vi "labHolo.vi"() -> ()   [LabVIEW 2023] (continued)
    tunnel: [w306] -> w9
    tunnel: w7 -> [w304]
    tunnel: w5 -> [w323]
    tunnel: w4 -> [w303]
    tunnel: w3 -> [w302]
    tunnel: w14 -> [w1060]
    tunnel: w12 -> [w1057]
    tunnel: w11 -> [w1056]
    tunnel: w10 -> [w1055]
    tunnel: w9 -> [w1054]
    frame #0 {
      w66 = T15 7 items=["Grayscale (U8)", "Grayscale (I16)", "Grayscale (SGL)", "Complex (CSG)", "RGB (U32)", "HSL (U32)", "RGB (U64)", "Grayscale (U16)"] ("Image Type")
      w68 = T15 4 items=["Grayscale (U8)", "Grayscale (I16)", "Grayscale (SGL)", "Complex (CSG)", "RGB (U32)", "HSL (U32)", "RGB (U64)", "Grayscale (U16)"] ("Image Type")
      # "Controls definition"
      n2 = Current VI's Path() -> (path=w133:path)
      n3 = Strip Path(path=w133) -> (stripped path=→"path":path)  [unwired: 1 out]
      n4 = case shown="\"16bits\", Default" "bit depth" {
        tunnel: [w152 w154] -> w117
        tunnel: [TRUE FALSE] -> w122
        frame "16bits", Default {
          w152 = T15 7 items=["Grayscale (U8)", "Grayscale (I16)", "Grayscale (SGL)", "Complex (CSG)", "RGB (U32)", "HSL (U32)", "RGB (U64)", "Grayscale (U16)"] ("Image Type")
        }
        frame "8bits" {
          w154 = T15 0 items=["Grayscale (U8)", "Grayscale (I16)", "Grayscale (SGL)", "Complex (CSG)", "RGB (U32)", "HSL (U32)", "RGB (U64)", "Grayscale (U16)"] ("Image Type")
        }
      }
      n5 = call "IMAQ Create"("Image Name"="monoHolo", "Image Type"=w66) -> ("New Image"=w65:T6)  [unwired: 3 in, 1 out]
      n6 = call "labHolo_path.vi"("sub folder or file (str)"="SupportFiles\\TestPatterns\\no_image.png") -> ("labHolo path"=w98:path)  [unwired: 1 in, 1 out]
      n7 = call "IMAQ Create"("Image Name"="holoSLM", "Image Type"=w68) -> ("New Image"=w63:T6)  [unwired: 3 in, 1 out]
      n8 = call "IMAQ Create"("Image Name"="holoMonitor", "Image Type"=w68) -> ("New Image"=w64:T6, "error out"=w67:errorcluster)  [unwired: 3 in]
      n9 = call "IMAQ Create"("Image Name"="Theo. beam", "Image Type"=w68) -> ("New Image"=w93:T6)  [unwired: 3 in, 1 out]
      n10 = call "positionManager.vi"("Display"=2, "Cluster"="2_posCluster") -> ("output cluster"=w107:cluster{i32, i32})  [unwired: 5 in, 2 out]
      n11 = call "positionManager.vi"("Display"=1, "Cluster"="1_posCluster") -> ("output cluster"=w106:cluster{i32, i32})  [unwired: 5 in, 2 out]
      n12 = call "initialize.vi"("14bits"=w122, "sys Python version"="3.9") -> ("session out"=w61:refnum<k35>, "available cameras"=w129:cluster{string[], string[]}, "error out"=w128:errorcluster)  [unwired: 2 in]
      "available\ncameras" <- w129
      n13 = case shown="1" "SLM_number" {
        tunnel: [w144 w146] -> w112
        tunnel: [w143 w148] -> w111
        tunnel: "1_posCluster" -> [w144 _]
        tunnel: "1_mainPos" -> [w143 _]
        tunnel: "2_posCluster" -> [_ w146]
        tunnel: "2_mainPos" -> [_ w148]
        tunnel: "SLM1 cluster" -> [w142 _]
        tunnel: "SLM2 cluster" -> [_ w147]
        tunnel: [w142 w147] -> w100
        tunnel: [w141 w145] -> w101
        tunnel: w107 -> [_ w145]
        tunnel: w106 -> [w141 _]
        frame 0, Default {
        }
        frame 1 {
        }
      }
      n14 = Unbundle(w129) -> (w114:string[])  [unwired: 1 out]
      n15 = local read "Selected Newport Device"() -> (w78:T1)
      n16 = call "IMAQ Create"("Image Name"="ROI image", "Image Type"=w117) -> ("New Image"=w116:T6)  [unwired: 3 in, 1 out]
      n17 = call "IMAQ Create"("Image Name"="Ref Image", "Image Type"=w117) -> ("New Image"=w119:T6)  [unwired: 3 in, 1 out]
      n18 = call "IMAQ Create"("Image Name"="CCD Image", "Image Type"=w117) -> ("New Image"=w120:T6)  [unwired: 3 in, 1 out]
      n19 = property on="Camera ID" class="Ring (strict)"("Strings []"=w114) -> ("Value"=w90:u16)  [unwired: 2 in, 2 out]
      n20 = Open Python Session(python version="3.9") -> (session out=w60:refnum<k35>)  [unwired: 2 in, 1 out]
      n21 = call "Connect Newport Instrument.vi"("Selected Device Cluster (INPUT)"=w78) -> ("error (duplicate)"=w77:errorcluster, "Device Connection Cluster"=w75:T16, "Selected Device Cluster (OUTPUT)"=w74:T1)  [unwired: 5 in, 3 out]
      n22 = property on="Zoom2Fit" class="Bool (strict)"("DisabledEnum"=T10."Disabled and Grayed Out" ("Disabled")) -> ()  [unwired: 2 in, 2 out]
      n23 = Bundle("New Image"=w65, "New Image"=w64, "New Image"=w63) -> (w62:T17)  [unwired: 1 in]
      n24 = Unbundle(w101) -> (→"Xpos":i32, →"Ypos":i32)
      n25 = Array Size(array=w114) -> (size(s)=w84:i32)
      n26 = case shown="No Error" w77 {
        tunnel: [w137 w140] -> w76
        tunnel: w75 -> [w137 _]
        tunnel: w74 -> [w136 _]
        tunnel: [w136 w138] -> w73
        frame No Error {
        }
        frame Error {
          n27 = call "Connect Newport Instrument.vi"("Selected Device Cluster (INPUT)"=T11 {"Found resources names"=["ASRL1::INSTR", "ASRL3::INSTR"], "Found interfaces names"=["ASRL1  (COM1 - Puerto de comunicaciones)", "ASRL3  (COM3 - USB Serial Port)"], "OK?"=FALSE, "Selected device"="", "Address"=0, "error"={"status"=TRUE, "code"=0, "source"=""}}) -> ("Device Connection Cluster"=w140:T16, "Selected Device Cluster (OUTPUT)"=w138:T1)  [unwired: 5 in, 4 out]
        }
      }
      "Selected Newport Device" <- w73
      n28 = Index Array(array=w114, index=0) -> (element=w115:string)
      n29 = local write "EnlargeCCD"(FALSE) -> ()
      n30 = case shown="\"Any\", Default" w115 {
        tunnel: w90 -> [_ _]
        tunnel: [FALSE TRUE] -> w89
        frame "Any", Default {
        }
        frame "NotFound" {
        }
      }
      n31 = call "rearrengeArray.vi"("array in"="exposures", "desired size"=w84) -> ("array out"=w82:dbl[])
      n32 = Not(x="Devel?") -> (.not. x?=w87:bool)
      n33 = call "rearrengeArray.vi"("array in"="FPSs", "desired size"=w84) -> ("array out"=w85:dbl[])
    }
    frame #1 {
      w187 = FALSE ("Visible")
      # "just in case, no image"
      # "CHANGE THIS!"
      # "Indicators (setting up)"
      n34 = And(x=w207, y=w206) -> (x .and. y?=w208:bool)
      n35 = Unbundle By Name(w248) -> ("1_Xcenter"=→"Xcenter":dbl, "1_Ycenter"=→"Ycenter":dbl, "1_Diam. X"=→"Diam. X":dbl, "1_Diam. Y"=→"Diam. Y":dbl, "1_Form fa."=→"Form fa.":dbl)
      n36 = for {
        N: w203 -> [_]
        tunnel: w222 -> [w289]
        tunnel: w221 -> [w288]
        tunnel: [w287] -> w220
        tunnel: [w286] -> w216 mode=indexing
        tunnel: [w285] -> w217 mode=indexing
        tunnel: [w283] -> w214 mode=indexing
        tunnel: [w282] -> w213
        tunnel: w211 -> [w281] mode=indexing
        tunnel: w212 -> [w280] mode=indexing
        tunnel: w207 -> [w276]
        i -> [w279]
        n37 = call "start.vi"("Not found"=w276, "Cam id"=w279, "error in (no error)"=w288, "Exposure (ms)"=w280, "FPS"=w281, "session in"=w289) -> ("error out"=w282:errorcluster, "cam attr."=w284:T18, "session out"=w287:refnum<k35>)  [unwired: 2 in]
        n38 = Unbundle By Name(w284) -> ("x"=w278:i32, "y"=w277:i32, "FPS"=w286:dbl, "Exposure"=w285:dbl)
        n39 = Bundle("x"=w278, "y"=w277) -> (w283:cluster{"x":i32, "y":i32})  [unwired: 1 in]
      }
      "Cam sizes" <- w214
      n40 = Unbundle By Name(w247) -> ("1_Xoffset"=w257:dbl, "1_Yoffset"=w256:dbl, "1_Xgros"=w255:dbl, "1_Ygros"=w254:dbl, "1_Xfine"=w253:dbl, "1_Yfine"=w252:dbl, "1_Xreverse"=w251:u16, "1_Yreverse"=w250:u16, "1_XYswap"=w249:u16)
      n41 = Increment(x=w201) -> (x+1=w202:u16)
      n42 = Unbundle By Name(w231) -> ("1_Radio"=w182:T7, "1_Trans"=w246:dbl, "1_Phase"=w245:dbl, "1_HoloCode"=w244:string, "1_Semi"=w243:bool, "1_Active"=w242:u16, "1_ModType"=w241:string, "1_Flip"=w240:string, "1_HoloNum"=w239:dbl, "1_key1"=w238:string, "1_value1"=w237:i64, "1_key2"=w236:string, "1_value2"=w159:i64, "1_Calibration file"=w158:string, "1_SLM brand"=w157:string)
      n43 = case shown="False" w208 {
        tunnel: [T10."Enabled" ("Disabled") T10."Disabled and Grayed Out" ("Disabled")] -> w200
        frame False {
        }
        frame True {
        }
      }
      n44 = Greater?(x=w202, y=w203) -> (0:w204:bool)
      n45 = call "CONEX-CC Get Stage Identifier v2.vi"("Connection Cluster in"=w194) -> ("Identifier"=→"ID":string, "Connection Cluster out"=w190:T16)  [unwired: 9 in]
      n46 = call "IMAQ ReadFile"("File Path"=w175, "Image"=w263) -> ("Image Out"=w262:T6)  [unwired: 5 in, 4 out]
      n47 = case shown="0, Default" w233 {
        tunnel: [u16 2 u16 1] -> w181
        tunnel: [u16 1 ("Display") u16 2 ("Display")] -> w174
        tunnel: [w293 w301] -> w172
        tunnel: w173 -> [w293 w300]
        tunnel: w171 -> [w292 w301]
        tunnel: [w292 w300] -> w156
        tunnel: [w291 w297] -> w163
        tunnel: w162 -> [w290 w297]
        tunnel: w161 -> [w291 w296]
        tunnel: [w290 w296] -> w160
        frame 0, Default {
        }
        frame 1 {
        }
      }
      n48 = property on="FPS" class="DigNum (strict)"("DisabledEnum"=w200) -> ()  [unwired: 2 in, 2 out]
      n49 = property on="bit depth" class="Enum (strict)"("DisabledEnum"=w200) -> ()  [unwired: 2 in, 2 out]
      n50 = property on="Gain" class="DigNum (strict)"("DisabledEnum"=w200) -> ()  [unwired: 2 in, 2 out]
      n51 = call "getSavePath.vi"("beam_name"=w226, "Polarizer"=w225, "Analyzer"=w224, "prefix"=w223, "suffix"=w264, "active"=w186) -> ("appended filename"=→"default filename":string)  [unwired: 9 in]
      n52 = property on="(1) Go to:" class="DigNum (strict)"("Caption.Text"=w196) -> ()  [unwired: 2 in, 2 out]
      n53 = property on="(2) Go to:" class="DigNum (strict)"("Caption.Text"=w196) -> ()  [unwired: 2 in, 2 out]
      n54 = property on="Step:" class="DigNum (strict)"("Caption.Text"=w196) -> ()  [unwired: 2 in, 2 out]
      n55 = property on="Raw position" class="DigNum (strict)"("Caption.Text"=w196) -> ()  [unwired: 2 in, 2 out]
      n56 = property on="Relative pos." class="DigNum (strict)"("Caption.Text"=w196) -> ()  [unwired: 2 in, 2 out]
      n57 = property on="Zero pos." class="DigNum (strict)"("Caption.Text"=w196) -> ()  [unwired: 2 in, 2 out]
      n58 = local write "Gain"(0.0 ("Gain")) -> ()
      n59 = case shown="False" w204 {
        frame False {
        }
        frame True {
          n60 = local write "Camera ID"(u16 0) -> ()
        }
      }
      n61 = local write "Xreverse"(w251) -> ()
      n62 = local write "Yreverse"(w250) -> ()
      n63 = local write "XYswap"(w249) -> ()
      n64 = local write "Xoffset"(w257) -> ()
      n65 = local write "Ygros"(w254) -> ()
      n66 = local write "Xfine"(w253) -> ()
      n67 = local write "Yoffset"(w256) -> ()
      n68 = local write "Xgros"(w255) -> ()
      n69 = local write "Yfine"(w252) -> ()
      n70 = property on="stop travel" class="Bool (strict)"("Visible"=w187, "Value"=w187) -> ()  [unwired: 2 in, 2 out]
      n71 = call "loadShowHolo.vi"("mainPos"=w160, "Python session"=w176, "Display"=w181, "error in (no error)"=w180, "prev. path"=w175, "SLM1 cluster"=w172, "holoImages"=w169) -> ("error out"=w177:errorcluster)  [unwired: 1 in, 3 out]
      n72 = property on="Exposure (ms)" class="DigNum (strict)"("DisabledEnum"=w200) -> ()  [unwired: 2 in, 2 out]
      n73 = property on="Camera ID" class="Ring (strict)"("DisabledEnum"=w200) -> ()  [unwired: 2 in, 2 out]
      n74 = local write "Radio"(w182) -> ()
      n75 = local write "Trans"(w246) -> ()
      n76 = local write "Phase"(w245) -> ()
      n77 = local write "HoloCode"(w244) -> ()
      n78 = local write "Semi"(w243) -> ()
      n79 = local write "Active"(w242) -> ()
      n80 = local write "ModType"(w241) -> ()
      n81 = local write "Flip"(w240) -> ()
      n82 = local write "HoloNum"(w239) -> ()
      n83 = local write "key1"(w238) -> ()
      n84 = local write "value1"(w237) -> ()
      n85 = local write "key2"(w236) -> ()
      n86 = local write "value2"(w159) -> ()
      n87 = local write "Calibration file"(w158) -> ()
      n88 = local write "SLM brand"(w157) -> ()
      n89 = call "CONEX-CC Get Positioner Error And Controller State v2.vi"("Connection Cluster in"=w190) -> ("Controller state"=→"Controller state":string, "Positioner error"=→"Positioner error":string, "Connection Cluster out"=w189:T16)  [unwired: 8 in]
      n90 = call "transAndPhaseManager.vi"("Trans in"=w267, "Phase in"=w266) -> ("Trans %"=→"T%":dbl, "Intensity"=→"Int":dbl, "T gl"=→"Tgl":dbl, "Phase Deg"=→"PhDeg":dbl, "Phase Rad"=→"PhRad":dbl)  [unwired: 9 in]
      n91 = Number To Decimal String(number=w234) -> (decimal integer string=→"1_HoloName":string)  [unwired: 1 in]
      n92 = call "loadShowHolo.vi"("mainPos"=w163, "Python session"=w176, "Display"=w174, "error in (no error)"=w177, "prev. path"=w175, "SLM1 cluster"=w156, "holoImages"=w169) -> ("error out"=w178:errorcluster, "appended path"=w170:path, "holo2show out"=→"monitor1" →"monitor2":T6)  [unwired: 1 in, 1 out]
      "CGH path" <- w170
      n93 = call "holoPathEditor.vi"("Display"=u16 0, "prev. Path"=w175, "input cluster"=w156) -> ("appended path"=w230:path)  [unwired: 5 in, 3 out]
      n94 = call "CONEX-CC Get Negative Software Limit v2.vi"("Connection Cluster in"=w189) -> ("Connection Cluster out"=w188:T16)  [unwired: 9 in, 1 out]
      n95 = control-ref of="help code"() -> (w183:refnum<vi>)
      n96 = Initialize Array(0.0 ("element"), w203) -> (w210:dbl[])
      n97 = Index Array(array=w217, index=w218) -> (element=w215:dbl)
      n98 = control-ref of="Available holograms:"() -> (w185:refnum<vi>)
      n99 = control-ref of="HoloCode"() -> (w184:refnum<vi>)
      n100 = Index Array(array=w216, index=w218) -> (element=w219:dbl)
      n101 = local write "exposures"(w217) -> ()
      n102 = local write "FPSs"(w216) -> ()
      n103 = call "CONEX-CC Get Positive Software Limit v2.vi"("Connection Cluster in"=w188) -> ("Connection Cluster out"=w197:T16)  [unwired: 9 in, 1 out]
      n104 = local write "Exposure (ms)"(w215) -> ()
      n105 = call "readImageIfExists.vi"("appended path"=w230, "Refnum in"=w232) -> ("Refnum out"=w199:T6)  [unwired: 8 in, 1 out]
      "theo. beam" <- w199
      n106 = local write "FPS"(w219) -> ()
      n107 = local write "gains"(w210) -> ()
      n108 = call "holoCodeOrHoloDir.vi"("Radio bottons"=w182, "HoloList Reff"=w185, "HoloHelp Reff"=w183, "HoloCode Reff"=w184) -> ()  [unwired: 8 in]
      n109 = control-ref of="Calibration file"() -> (w155:refnum<vi>)
      n110 = local write "take reff"(FALSE ("take reff")) -> ()
      n111 = call "CONEX-CC Get Velocity v2.vi"("Connection Cluster in"=w197) -> ("Connection Cluster out"=w195:T16)  [unwired: 8 in, 2 out]
      n112 = call "fill_calibration_options.vi"("ComboBox in"=w155) -> ()  [unwired: 11 in]
      "Reff alert" <- FALSE ("Boolean")
    }
    frame #2 {
      n113 = Obtain Notifier(name (unnamed)="suffix", notification data type="") -> (notifier out=w310:refnum<notifier>)  [unwired: 2 in, 2 out]
      n114 = Obtain Notifier(name (unnamed)="filename", notification data type="") -> (notifier out=w309:refnum<notifier>)  [unwired: 2 in, 2 out]
      n115 = Obtain Notifier(name (unnamed)="Rel. Pos", notification data type=0.0) -> (notifier out=w306:refnum<notifier>)  [unwired: 2 in, 2 out]
      n116 = Obtain Notifier(name (unnamed)="step_done", notification data type="") -> (notifier out=w311:refnum<notifier>)  [unwired: 2 in, 2 out]
      n117 = node-c288() -> (w321:T12)  [unwired: 2 in, 1 out]
      n118 = while {
        tunnel: w310 -> [w334]
        tunnel: w311 -> [w333]
        tunnel: w309 -> [w332]
        tunnel: w306 -> [w331]
        stop <- w335 stop-if-true
        n119 = local read "Travel"() -> (w336:bool)
        n120 = case shown="True" w336 {
          tunnel: w334 -> [_ w357]
          tunnel: w333 -> [_ w356]
          tunnel: w332 -> [_ w338]
          tunnel: w331 -> [_ w337]
          frame False {
          }
          frame True {
            w345 = FALSE ("Visible")
            # "Ending"
            # "Checking"
            n121 = property on="stop travel" class="Bool (strict)"("Visible"=TRUE, "DisabledEnum"=T10."Enabled" ("Disabled"), "Value"=FALSE ("stop travel")) -> (error out=w352:errorcluster)  [unwired: 2 in, 1 out]
            n122 = local read "Relative pos."() -> (w349:dbl)
            n123 = local read "(2) Go to:"() -> (w343:dbl)
            n124 = local read "Last mov."() -> (w350:u16)
            n125 = local read "(1) Go to:"() -> (w351:dbl)
            n126 = local read "Step:"() -> (w341:dbl)
            n127 = Divide(x=w341, y=2.0) -> (x/y=w339:dbl)
            n128 = call "checkInitialPosition.vi"("Last mov."=w350, "error in (no error)"=w352, "Step"=w341, "Initial pos"=w351, "Current pos"=w349) -> ("error out"=w348:errorcluster, "go"=w344:bool)  [unwired: 5 in]
            n129 = Subtract(x=w343, y=w339) -> (x-y=w342:dbl)
            n130 = case shown="True" w344 {
              tunnel: w357 -> [_ w365]
              tunnel: w356 -> [_ w364]
              tunnel: w348 -> [w358 w363]
              tunnel: [w358 w362] -> w347
              tunnel: w342 -> [_ w361]
              tunnel: w338 -> [_ w360]
              tunnel: w337 -> [_ w359]
              frame False {
              }
              frame True {
                n131 = while {
                  tunnel: w365 -> [w381]
                  tunnel: w364 -> [w370]
                  tunnel: w363 -> [w374]
                  tunnel: [w368] -> w362
                  tunnel: w361 -> [w379]
                  tunnel: w360 -> [w375]
                  tunnel: w359 -> [w372]
                  i -> [w380]
                  stop <- w384 stop-if-true
                  # "Travel"
                  n132 = local read "SaveTravel"() -> (w383:bool)
                  n133 = Wait on Notification with Notifier History(0:w372, 1:TRUE ("ignore previous (F)"), 3:w374) -> (9:w371:dbl, 11:w373:errorcluster)  [unwired: 1 in, 2 out]
                  n134 = case shown="True" w383 {
                    tunnel: w373 -> [w385 w391]
                    tunnel: [w385 w386] -> w376
                    tunnel: w381 -> [_ w389]
                    tunnel: w371 -> [_ w393]
                    tunnel: w375 -> [_ w388]
                    frame False {
                    }
                    frame True {
                      n135 = local read "Units"() -> (w394:string)
                      n136 = call "getZsuffix.vi"("Units"=w394, "Zposition"=w393) -> ("String"=w390:string)  [unwired: 9 in]
                      n137 = Send Notification(notification=w390, notifier=w389, error in (no error)=w391) -> (error out=w392:errorcluster)  [unwired: 1 out]
                      n138 = property on="Save" class="Bool (strict)"(error in=w392, "Val(Sgnl)"=TRUE ("Value (Signaling)")) -> (error out=w387:errorcluster)  [unwired: 1 in, 1 out]
                      n139 = Wait on Notification with Notifier History(0:w388, 3:w387) -> (11:w386:errorcluster)  [unwired: 2 in, 3 out]
                    }
                  }
                  n140 = Greater Or Equal?(x=w371, y=w379) -> (x >= y?=w377:bool)
                  n141 = property on="step forward" class="Bool (strict)"(error in=w376, "Val(Sgnl)"=TRUE ("Value (Signaling)")) -> (error out=w369:errorcluster)  [unwired: 1 in, 1 out]
                  n142 = Or(x="stop travel", y=w377) -> (x .or. y?=w384:bool)
                  n143 = call "waitNotifierWithTime.vi"("min wait in ms (500)"=u32 1000 ("min wait in ms (300)"), "error in (no error)"=w369, "Notifier in"=w370) -> ("error out"=w368:errorcluster)  [unwired: 6 in, 2 out]
                  "Travel Count" <- w380
                }
              }
            }
            n144 = property on="stop travel" class="Bool (strict)"(error in=w347, "Visible"=w345, "Value"=w345) -> (error out=w346:errorcluster)  [unwired: 1 in, 1 out]
            n145 = property on="Travel" class="Bool (strict)"(error in=w346, "Value"=w345) -> ()  [unwired: 1 in, 2 out]
          }
        }
        n146 = local read "Parada Total"() -> (w335:bool)
      }
      n147 = while {
        tunnel: w324 -> [w563]
        shift-right: [w562] -> _
        shift-left: w323 -> [w561]
        shift-right: [w559] -> _
        shift-left: w303 -> [w558]
        shift-right: [w556] -> _
        shift-left: w322 -> [w557]
        tunnel: w304 -> [w555]
        tunnel: w302 -> [w554]
        stop <- w564 stop-if-true
        # "HoloImages"
        # "SLM control"
        # "CGH path"
        # "Theo"
        n148 = event shown="[1] \"Radio\", \"Trans\", \"HoloNum\", \"ModType\", \"Semi\", \"Active\", \"value1\", \"key1\", \"key2\", \"Phase\", \"Flip\", \"HoloCode\", \"TrueHolo?\", \"Calibration file\", \"SLM brand\": Value Change" {
          selector: _ -> [_ _ _ _ _ _ _ _]
          dyn-events: _ -> [_ _ _ _ _ _ _ _]
          timeout: _ -> [_ _ _ _ _ _ _ _]
          tunnel: w557 -> [w566 w585 w661 w669 w724 w786 _ w867]
          tunnel: [_ _ _ _ _ _ _ w868] -> w564
          tunnel: w563 -> [_ _ _ _ _ _ _ _]
          tunnel: [w565 w583 _ w667 w722 w784 w824 w865] -> w562
          tunnel: w561 -> [w565 w590 _ w667 w722 w784 w824 w865]
          tunnel: [_ w584 _ _ _ _ w828 _] -> w560
          tunnel: [w567 w586 w660 w668 w723 w785 w827 w866] -> w559
          tunnel: w558 -> [w567 w587 _ w668 w723 w785 w826 w866]
          tunnel: [w566 w585 w661 w669 w724 w786 w825 w867] -> w556
          tunnel: w555 -> [_ w573 _ _ _ _ _ w864]
          tunnel: w554 -> [_ w572 _ _ _ _ w822 _]
          event Timeout {
            n149 = event-data() -> ()  [unwired: 1 in, 3 out]
          }
          event "Radio", "Trans", "HoloNum", "ModType", "Semi", "Active", "value1", "key1", "key2", "Phase", "Flip", "HoloCode", "TrueHolo?", "Calibration file", "SLM brand": Value Change {
            # "Display = #item + 1"
            # "Old"
            # "New"
            n150 = event-data() -> ("CtlRef"=w588:refnum<vi>, "OldVal"=w593:variant, "NewVal"=w589:variant)  [unwired: 1 in]
            n151 = case shown="0, Default" w585 {
              tunnel: [w598 w600] -> w570
              tunnel: [w597 w599] -> w571
              frame 0, Default {
                n152 = local read "SLM1 cluster"() -> (w598:T2)
                n153 = local read "1_mainPos"() -> (w597:T3)
              }
              frame 1 {
                n154 = local read "SLM2 cluster"() -> (w600:T2)
                n155 = local read "2_mainPos"() -> (w599:T3)
              }
            }
            n156 = property class="Ctl"(reference=w588) -> ("Label.Text"=w594:string)  [unwired: 1 in, 2 out]
            n157 = call "updateHoloBundle.vi"("NewValue"=w589, "input cluster"=w570, "CtlRef"=w588) -> ("output cluster"=w569:T19)  [unwired: 7 in, 1 out]
            n158 = local read "TrueHolo?"() -> (w568:bool)
            n159 = Increment(x=w585) -> (x+1=w592:u16)
            n160 = call "loadShowHolo.vi"("mainPos"=w571, "True hologram?"=w568, "Python session"=w573, "Display"=w592, "error in (no error)"=w590, "prev. path"=w587, "SLM1 cluster"=w569, "holoImages"=w572) -> ("error out"=w583:errorcluster, "path exist"=w591:bool, "appended path"=w586:path, "holo2show out"=w584:T6)
            n161 = case shown="\"Any\", Default" w594 {
              tunnel: w593 -> [w602 w608 _ w614 _ w625 w631 w638 _ _]
              tunnel: w589 -> [_ _ _ _ w623 _ _ w636 w653 w657]
              tunnel: w591 -> [w601 w607 _ w613 _ w624 w630 w637 _ _]
              frame "HoloNum" {
                n162 = case shown="True" w601 {
                  tunnel: w602 -> [w603 _]
                  frame False {
                    n163 = feedback #1() -> (w604:dbl)  [unwired: 1 in]
                    n164 = Variant To Data(type=w604, Variant=w603) -> (data=w606:dbl)  [unwired: 1 in, 1 out]
                    n165 = property on="HoloNum" class="DigNum (strict)"("Value"=w606) -> ("Value"=w605:dbl)  [unwired: 2 in, 2 out]
                    n166 = feedback-in #1(w605) -> ()
                  }
                  frame True {
                  }
                }
              }
              frame "ParamStr" {
                n167 = case shown="True" w607 {
                  tunnel: w608 -> [w609 _]
                  frame False {
                    n168 = feedback #2() -> (w610:string)  [unwired: 1 in]
                    n169 = Variant To Data(type=w610, Variant=w609) -> (data=w612:string)  [unwired: 1 in, 1 out]
                    n170 = property on="key1" class="Str"("Value"=w612) -> ("Value"=w611:string)  [unwired: 2 in, 2 out]
                    n171 = feedback-in #2(w611) -> ()
                  }
                  frame True {
                  }
                }
              }
              frame "Any", Default {
              }
              frame "ParamVal" {
                n172 = case shown="True" w613 {
                  tunnel: w614 -> [w615 _]
                  frame False {
                    n173 = feedback #3() -> (w616:i64)  [unwired: 1 in]
                    n174 = Variant To Data(type=w616, Variant=w615) -> (data=w618:i64)  [unwired: 1 in, 1 out]
                    n175 = property on="value1" class="DigNum (strict)"("Value"=w618) -> ("Value"=w617:i64)  [unwired: 2 in, 2 out]
                    n176 = feedback-in #3(w617) -> ()
                  }
                  frame True {
                  }
                }
              }
              frame "Active" {
                n177 = Variant To Data(type=0, Variant=w623) -> (data=w619:i32)  [unwired: 1 in, 1 out]
                n178 = Not Equal?(x=u16 0, y=w619) -> (x != y?=w620:bool)
                n179 = property on="Active" class="Ring (strict)"("Blinking"=w620) -> ()  [unwired: 2 in, 2 out]
              }
              frame "ParamAux" {
                n180 = case shown="False" w624 {
                  tunnel: w625 -> [w626 _]
                  frame False {
                    n181 = feedback #4() -> (w627:string)  [unwired: 1 in]
                    n182 = Variant To Data(type=w627, Variant=w626) -> (data=w629:string)  [unwired: 1 in, 1 out]
                    n183 = property on="key2" class="Str"("Value"=w629) -> ("Value"=w628:string)  [unwired: 2 in, 2 out]
                    n184 = feedback-in #4(w628) -> ()
                  }
                  frame True {
                  }
                }
              }
              frame "ModType" {
                n185 = case shown="False" w630 {
                  tunnel: w631 -> [w633 _]
                  frame False {
                    n186 = feedback #5() -> (w635:string)  [unwired: 1 in]
                    n187 = Variant To Data(type=w635, Variant=w633) -> (data=w632:string)  [unwired: 1 in, 1 out]
                    n188 = property on="ModType" class="CmbBox"("Value"=w632) -> ("Value"=w634:string)  [unwired: 2 in, 2 out]
                    n189 = feedback-in #5(w634) -> ()
                  }
                  frame True {
                  }
                }
              }
              frame "Radio" {
                n190 = case shown="True" w637 {
                  tunnel: w638 -> [w641 _]
                  tunnel: w636 -> [_ w647]
                  frame False {
                    n191 = Variant To Data(type=0, Variant=w641) -> (data=w639:i32)  [unwired: 1 in, 1 out]
                    n192 = local write "Radio"(w639) -> ()
                  }
                  frame True {
                    n193 = Variant To Data(type=0, Variant=w647) -> (data=w645:i32)  [unwired: 1 in, 1 out]
                    n194 = control-ref of="help code"() -> (w642:refnum<vi>)
                    n195 = control-ref of="HoloCode"() -> (w643:refnum<vi>)
                    n196 = control-ref of="Available holograms:"() -> (w644:refnum<vi>)
                    n197 = call "holoCodeOrHoloDir.vi"("Radio bottons"=w645, "HoloList Reff"=w644, "HoloHelp Reff"=w642, "HoloCode Reff"=w643) -> ()  [unwired: 8 in]
                  }
                }
              }
              frame "Trans" {
                n198 = Variant To Data(type=0.0, Variant=w653) -> (data=w651:dbl)  [unwired: 1 in, 1 out]
                n199 = call "transAndPhaseManager.vi"("Trans in"=w651) -> ("Trans %"=w650:dbl, "Intensity"=w649:dbl, "T gl"=w648:dbl)  [unwired: 10 in, 2 out]
                n200 = local write "T%"(w650) -> ()
                n201 = local write "Int"(w649) -> ()
                n202 = local write "Tgl"(w648) -> ()
              }
              frame "Phase" {
                n203 = Variant To Data(type=0.0, Variant=w657) -> (data=w654:dbl)  [unwired: 1 in, 1 out]
                n204 = call "transAndPhaseManager.vi"("Phase in"=w654) -> ("Phase Deg"=w656:dbl, "Phase Rad"=w655:dbl)  [unwired: 10 in, 3 out]
                n205 = local write "PhDeg"(w656) -> ()
                n206 = local write "PhRad"(w655) -> ()
              }
            }
            n207 = case shown="0, Default" w585 {
              tunnel: w569 -> [w595 w596]
              frame 0, Default {
                n208 = local write "SLM1 cluster"(w595) -> ()
              }
              frame 1 {
                n209 = local write "SLM2 cluster"(w596) -> ()
              }
            }
            n210 = local read "Radio"() -> (w576:T7)
            n211 = local read "Active"() -> (w582:u16)
            n212 = call "enableDisableSLMbuttons.vi"("Active"=w582, "Radio"=w576) -> ("Semi"=w577:T10, "ModType"=w578:T10, "Phase"=w579:T10, "Trans"=w580:T10, "HoloCode"=w574:T10, "PrefabrHolo"=w581:T10, "just ON/OFF"=w575:T10)  [unwired: 3 in]
            n213 = property on="Flip" class="CmbBox"("DisabledEnum"=w575) -> ()  [unwired: 2 in, 2 out]
            n214 = property on="Radio" class="RadioBtnsControl (strict)"("DisabledEnum"=w575) -> ()  [unwired: 2 in, 2 out]
            n215 = property on="HoloNum" class="DigNum (strict)"("DisabledEnum"=w581) -> ()  [unwired: 2 in, 2 out]
            n216 = property on="key2" class="Str"("DisabledEnum"=w581) -> ()  [unwired: 2 in, 2 out]
            n217 = property on="Xoffset" class="DigNum (strict)"("DisabledEnum"=w575) -> ()  [unwired: 2 in, 2 out]
            n218 = property on="Sync SLMs" class="Bool"("DisabledEnum"=w575) -> ()  [unwired: 2 in, 2 out]
            n219 = property on="ModType" class="CmbBox"("DisabledEnum"=w578) -> ()  [unwired: 2 in, 2 out]
            n220 = property on="Trans" class="Slide (strict)"("DisabledEnum"=w580) -> ()  [unwired: 2 in, 2 out]
            n221 = property on="setXi" class="Bool (strict)"("DisabledEnum"=w575) -> ()  [unwired: 2 in, 2 out]
            n222 = property on="key1" class="Str"("DisabledEnum"=w581) -> ()  [unwired: 2 in, 2 out]
            n223 = property on="value1" class="DigNum (strict)"("DisabledEnum"=w581) -> ()  [unwired: 2 in, 2 out]
            n224 = property on="Yoffset" class="DigNum (strict)"("DisabledEnum"=w575) -> ()  [unwired: 2 in, 2 out]
            n225 = property on="XYswap" class="Ring (strict)"("DisabledEnum"=w575) -> ()  [unwired: 2 in, 2 out]
            n226 = property on="Phase" class="Slide (strict)"("DisabledEnum"=w579) -> ()  [unwired: 2 in, 2 out]
            n227 = property on="T%" class="DigNum (strict)"("DisabledEnum"=w580) -> ()  [unwired: 2 in, 2 out]
            n228 = property on="setXf" class="Bool (strict)"("DisabledEnum"=w575) -> ()  [unwired: 2 in, 2 out]
            n229 = property on="Xgros" class="Slide (strict)"("DisabledEnum"=w575) -> ()  [unwired: 2 in, 2 out]
            n230 = property on="Semi" class="Bool (strict)"("DisabledEnum"=w577) -> ()  [unwired: 2 in, 2 out]
            n231 = property on="Xreverse" class="Ring (strict)"("DisabledEnum"=w575) -> ()  [unwired: 2 in, 2 out]
            n232 = property on="PhDeg" class="DigNum (strict)"("DisabledEnum"=w579) -> ()  [unwired: 2 in, 2 out]
            n233 = property on="setYi" class="Bool (strict)"("DisabledEnum"=w575) -> ()  [unwired: 2 in, 2 out]
            n234 = property on="Tgl" class="DigNum (strict)"("DisabledEnum"=w580) -> ()  [unwired: 2 in, 2 out]
            n235 = property on="Ygros" class="Slide (strict)"("DisabledEnum"=w575) -> ()  [unwired: 2 in, 2 out]
            n236 = property on="Yreverse" class="Ring (strict)"("DisabledEnum"=w575) -> ()  [unwired: 2 in, 2 out]
            n237 = property on="setYf" class="Bool (strict)"("DisabledEnum"=w575) -> ()  [unwired: 2 in, 2 out]
            n238 = property on="PhRad" class="DigNum (strict)"("DisabledEnum"=w579) -> ()  [unwired: 2 in, 2 out]
            n239 = property on="Int" class="DigNum (strict)"("DisabledEnum"=w580) -> ()  [unwired: 2 in, 2 out]
            n240 = property on="Xfine" class="Slide (strict)"("DisabledEnum"=w575) -> ()  [unwired: 2 in, 2 out]
            n241 = property on="help code" class="Bool"("DisabledEnum"=w574) -> ()  [unwired: 2 in, 2 out]
            n242 = property on="HoloCode" class="Str"("DisabledEnum"=w574) -> ()  [unwired: 2 in, 2 out]
            n243 = property on="doCenter" class="Bool (strict)"("DisabledEnum"=w575) -> ()  [unwired: 2 in, 2 out]
            n244 = property on="Yfine" class="Slide (strict)"("DisabledEnum"=w575) -> ()  [unwired: 2 in, 2 out]
          }
          event "Available holograms:": Value Change {
            n245 = event-data() -> ("NewVal"=w665:i32)  [unwired: 1 in, 5 out]
            n246 = property on="Available holograms:" class="LstBox (strict)"() -> ("Item Names"=w666:string[])  [unwired: 2 in, 2 out]
            n247 = Index Array(array=w666, index=w665) -> (element=w663:string)
            n248 = Concatenate Strings("..\\Holograms\\" ("string"), w663) -> (w664:string)
            n249 = call "labHolo_path.vi"("sub folder or file (str)"=w664) -> ("labHolo path"=w660:path)  [unwired: 1 in, 1 out]
            n250 = property on="Radio" class="RadioBtnsControl (strict)"("Val(Sgnl)"=T7."No Selection" ("Radio")) -> ()  [unwired: 2 in, 2 out]
          }
          event "Xoffset", "Yoffset", "Xgros", "Ygros", "Xfine", "Yfine", "doCenter": Value Change {
            n251 = event-data() -> ("CtlRef"=w672:refnum<vi>, "NewVal"=w671:variant)  [unwired: 1 in, 1 out]
            n252 = local write "doCenter"(FALSE ("doCenter")) -> ()
            n253 = case shown="1" w669 {
              tunnel: [w681 w682] -> w673
              frame 0, Default {
                n254 = local read "1_posCluster"() -> (w681:T4)
              }
              frame 1 {
                n255 = local read "2_posCluster"() -> (w682:T4)
              }
            }
            n256 = property class="Ctl"(reference=w672) -> ("Label.Text"=w677:string)  [unwired: 1 in, 2 out]
            n257 = case shown="\"Any\", Default" w677 {
              tunnel: w673 -> [w687 w692 w697 w702 w707 w712 w716 w721]
              tunnel: w671 -> [w686 w691 w696 w701 w706 w711 _ _]
              tunnel: [w683 w688 w693 w698 w703 w708 w715 w721] -> w678
              frame "Xoffset" {
                n258 = Variant To Data(type=0.0, Variant=w686) -> (data=w685:dbl)  [unwired: 1 in, 1 out]
                n259 = Bundle By Name(cluster=w687, "1_Xoffset"=w685) -> (w683:T4)
              }
              frame "Yoffset" {
                n260 = Variant To Data(type=0.0, Variant=w691) -> (data=w689:dbl)  [unwired: 1 in, 1 out]
                n261 = Bundle By Name(cluster=w692, "1_Yoffset"=w689) -> (w688:T4)
              }
              frame "Xgros" {
                n262 = Variant To Data(type=0.0, Variant=w696) -> (data=w694:dbl)  [unwired: 1 in, 1 out]
                n263 = Bundle By Name(cluster=w697, "1_Xgros"=w694) -> (w693:T4)
              }
              frame "Ygros" {
                n264 = Variant To Data(type=0.0, Variant=w701) -> (data=w699:dbl)  [unwired: 1 in, 1 out]
                n265 = Bundle By Name(cluster=w702, "1_Ygros"=w699) -> (w698:T4)
              }
              frame "Xfine" {
                n266 = Variant To Data(type=0.0, Variant=w706) -> (data=w704:dbl)  [unwired: 1 in, 1 out]
                n267 = Bundle By Name(cluster=w707, "1_Xfine"=w704) -> (w703:T4)
              }
              frame "Yfine" {
                n268 = Variant To Data(type=0.0, Variant=w711) -> (data=w709:dbl)  [unwired: 1 in, 1 out]
                n269 = Bundle By Name(cluster=w712, "1_Yfine"=w709) -> (w708:T4)
              }
              frame "doCenter" {
                n270 = local read "Xcenter"() -> (w720:dbl)
                n271 = local read "Ycenter"() -> (w718:dbl)
                n272 = local read "Xpos"() -> (w719:i32)
                n273 = local read "Ypos"() -> (w717:i32)
                n274 = call "centerHolo.vi"("posCluster"=w716, "Ypos"=w717, "Ycenter"=w718, "Xpos"=w719, "Xcenter"=w720) -> ("new Y gros"=w713:dbl, "new X gros"=w714:dbl)  [unwired: 4 in]
                n275 = Bundle By Name(cluster=w716, "1_Xgros"=w714, "1_Ygros"=w713) -> (w715:T4)
                n276 = local write "Xgros"(w714) -> ()
                n277 = local write "Ygros"(w713) -> ()
              }
              frame "Any", Default {
              }
            }
            n278 = case shown="1" w669 {
              tunnel: w678 -> [w679 w680]
              frame 0, Default {
                n279 = local write "1_posCluster"(w679) -> ()
              }
              frame 1 {
                n280 = local write "2_posCluster"(w680) -> ()
              }
            }
            n281 = Increment(x=w669) -> (x+1=w676:u16)
            n282 = call "positionManager.vi"("Display"=w676, "Cluster"=w678) -> ("Y position out"=w675:i32, "X position out"=w674:i32)  [unwired: 5 in, 1 out]
            n283 = local write "Xpos"(w674) -> ()
            n284 = local write "Ypos"(w675) -> ()
          }
          event "Xreverse", "Yreverse", "XYswap": Value Change {
            n285 = event-data() -> ("CtlRef"=w725:refnum<vi>, "NewVal"=w726:u16)  [unwired: 1 in, 1 out]
            n286 = case shown="1" w724 {
              tunnel: [w737 w739] -> w728
              tunnel: [w736 w738] -> w730
              frame 0, Default {
                n287 = local read "1_posCluster"() -> (w737:T4)
                n288 = local read "1_mainPos"() -> (w736:T3)
              }
              frame 1 {
                n289 = local read "2_posCluster"() -> (w739:T4)
                n290 = local read "2_mainPos"() -> (w738:T3)
              }
            }
            n291 = property class="Ring (strict)"(reference=w725) -> ("Label.Text"=w727:string)  [unwired: 1 in, 2 out]
            n292 = case shown="\"XYswap\"" w727 {
              tunnel: [w761 w763 w773 w776] -> w729
              tunnel: w728 -> [w760 w763 w772 w777]
              tunnel: w726 -> [w755 _ w765 w775]
              tunnel: w730 -> [w749 w762 w764 w774]
              tunnel: [w748 w762 w764 w774] -> w731
              frame "XYswap" {
                n293 = Unbundle By Name(w760) -> ("1_Xoffset"=w757:dbl, "1_Yoffset"=w759:dbl, "1_Xgros"=w756:dbl, "1_Ygros"=w758:dbl, "1_Xfine"=w744:dbl, "1_Yfine"=w747:dbl, "1_Xreverse"=w740:u16, "1_Yreverse"=w741:u16)
                n294 = Unbundle By Name(w749) -> ("1_Xcenter"=w746:dbl, "1_Ycenter"=w745:dbl)
                n295 = local write "Xcenter"(w745) -> ()
                n296 = local write "Ycenter"(w746) -> ()
                n297 = property on="Xoffset" class="DigNum (strict)"("Val(Sgnl)"=w759) -> (error out=w754:errorcluster)  [unwired: 2 in, 1 out]
                n298 = Bundle By Name(cluster=w760, "1_XYswap"=w755, "1_Xoffset"=w759, "1_Yoffset"=w757, "1_Xgros"=w758, "1_Ygros"=w756, "1_Xfine"=w747, "1_Yfine"=w744, "1_Xreverse"=w741, "1_Yreverse"=w740) -> (w761:T4)
                n299 = Bundle By Name(cluster=w749, "1_Ycenter"=w746, "1_Xcenter"=w745) -> (w748:T3)
                n300 = property on="Yoffset" class="DigNum (strict)"(error in=w754, "Val(Sgnl)"=w757) -> (error out=w751:errorcluster)  [unwired: 1 in, 1 out]
                n301 = property on="Xgros" class="Slide (strict)"(error in=w751, "Val(Sgnl)"=w758) -> (error out=w753:errorcluster)  [unwired: 1 in, 1 out]
                n302 = property on="Ygros" class="Slide (strict)"(error in=w753, "Val(Sgnl)"=w756) -> (error out=w750:errorcluster)  [unwired: 1 in, 1 out]
                n303 = property on="Xfine" class="Slide (strict)"(error in=w750, "Val(Sgnl)"=w747) -> (error out=w752:errorcluster)  [unwired: 1 in, 1 out]
                n304 = property on="Yfine" class="Slide (strict)"(error in=w752, "Val(Sgnl)"=w744) -> (error out=w743:errorcluster)  [unwired: 1 in, 1 out]
                n305 = property on="Xreverse" class="Ring (strict)"(error in=w743, "Value"=w741) -> (error out=w742:errorcluster)  [unwired: 1 in, 1 out]
                n306 = property on="Yreverse" class="Ring (strict)"(error in=w742, "Value"=w740) -> ()  [unwired: 1 in, 2 out]
              }
              frame "Any", Default {
              }
              frame "Xreverse" {
                w769 = -1
                n307 = Unbundle By Name(w772) -> ("1_Xgros"=w770:dbl, "1_Xfine"=w771:dbl)
                n308 = Multiply(x=w769, y=w770) -> (x*y=w768:dbl)
                n309 = Multiply(x=w771, y=w769) -> (x*y=w766:dbl)
                n310 = property on="Xgros" class="Slide (strict)"("Val(Sgnl)"=w768) -> (error out=w767:errorcluster)  [unwired: 2 in, 1 out]
                n311 = Bundle By Name(cluster=w772, "1_Xgros"=w768, "1_Xfine"=w766, "1_Xreverse"=w765) -> (w773:T4)
                n312 = property on="Xfine" class="Slide (strict)"(error in=w767, "Val(Sgnl)"=w766) -> ()  [unwired: 1 in, 2 out]
              }
              frame "Yreverse" {
                w781 = -1